vi "SaccadeAnalyser - Main.vi"(8 "error in (no error)":errorcluster, 11 "Data IN":T3={"Impulse Positions"=[{"Start"=5471, "End"=5813, "Impulse Plane"=enum."Yaw", "Impulse Direction +ve?"=FALSE, "Time offset"=0, "Amplitude offset"=0.0}, {"Start"=6974, "End"=7325, "Impulse Plane"=enum."Yaw", "Impulse Direction +ve?"=TRUE, "Time offset"=0, "Amplitude offset"=0.0}, {"Start"=7641, "End"=7980, "Impulse Plane"=enum."Yaw", "Impulse Direction +ve?"=FALSE, "Time offset"=0, "Amplitude offset"=0.0}, {"Start"=9060, "End"=9400, "Impulse Plane"=enum."Yaw", "Impulse Direction +ve?"=FALSE, "Time offset"=0, "Amplitude offset"=0.0}, {"Start"=9938, "End"=10282, "Impulse Plane"=enum."Yaw", "Impulse Direction +ve?"=FALSE, "Time offset"=0, "Amplitude offset"=0.0}, {"Start"=10800, "End"=11142, "Impulse Plane"=enum."Yaw", "Impulse Direction +ve?"=FALSE, "Time offset"=0, "Amplitude offset"=0.0}, {"Start"=11602, "End"=11942, "Impulse Plane"=enum."Yaw", "Impulse Direction +ve?"=TRUE, "Time offset"=0, "Amplitude offset"=0.0}, {"Start"=12449, "End"=12790, "Impulse Plane"=enum."Yaw", "Impulse Direction +ve?"=TRUE, "Time offset"=0, "Amplitude offset"=0.0}, {"Start"=13310, "End"=13653, "Impulse Plane"=enum."Yaw", "Impulse Direction +ve?"=TRUE, "Time offset"=0, "Amplitude offset"=0.0}, {"Start"=14191, "End"=14535, "Impulse Plane"=enum."Yaw", "Impulse Direction +ve?"=TRUE, "Time offset"=0, "Amplitude offset"=0.0}, {"Start"=15040, "End"=15380, "Impulse Plane"=enum."Yaw", "Impulse Direction +ve?"=FALSE, "Time offset"=0, "Amplitude offset"=0.0}, {"Start"=16780, "End"=17124, "Impulse Plane"=enum."Yaw", "Impulse Direction +ve?"=TRUE, "Time offset"=0, "Amplitude offset"=0.0}, {"Start"=17572, "End"=17913, "Impulse Plane"=enum."Yaw", "Impulse Direction +ve?"=FALSE, "Time offset"=0, "Amplitude offset"=0.0}, {"Start"=18369, "End"=18713, "Impulse Plane"=enum."Yaw", "Impulse Direction +ve?"=FALSE, "Time offset"=0, "Amplitude offset"=0.0}, {"Start"=19174, "End"=19519, "Impulse Plane"=enum."Yaw", "Impulse Direction +ve?"=FALSE, "Time offset"=0, "Amplitude offset"=0.0}, {"Start"=19928, "End"=20270, "Impulse Plane"=enum."Yaw", "Impulse Direction +ve?"=TRUE, "Time offset"=0, "Amplitude offset"=0.0}, {"Start"=20762, "End"=21121, "Impulse Plane"=enum."Yaw", "Impulse Direction +ve?"=FALSE, "Time offset"=0, "Amplitude offset"=0.0}, {"Start"=21554, "End"=21888, "Impulse Plane"=enum."Yaw", "Impulse Direction +ve?"=FALSE, "Time offset"=0, "Amplitude offset"=0.0}, {"Start"=22293, "End"=22639, "Impulse Plane"=enum."Yaw", "Impulse Direction +ve?"=TRUE, "Time offset"=0, "Amplitude offset"=0.0}, {"Start"=23109, "End"=23464, "Impulse Plane"=enum."Yaw", "Impulse Direction +ve?"=TRUE, "Time offset"=0, "Amplitude offset"=0.0}, {"Start"=23868, "End"=24215, "Impulse Plane"=enum."Yaw", "Impulse Direction +ve?"=TRUE, "Time offset"=0, "Amplitude offset"=0.0}, {"Start"=24643, "End"=24992, "Impulse Plane"=enum."Yaw", "Impulse Direction +ve?"=FALSE, "Time offset"=0, "Amplitude offset"=0.0}, {"Start"=25685, "End"=26023, "Impulse Plane"=enum."Yaw", "Impulse Direction +ve?"=FALSE, "Time offset"=0, "Amplitude offset"=0.0}, {"Start"=26431, "End"=26768, "Impulse Plane"=enum."Yaw", "Impulse Direction +ve?"=FALSE, "Time offset"=0, "Amplitude offset"=0.0}, {"Start"=27251, "End"=27595, "Impulse Plane"=enum."Yaw", "Impulse Direction +ve?"=FALSE, "Time offset"=0, "Amplitude offset"=0.0}, {"Start"=28832, "End"=29180, "Impulse Plane"=enum."Yaw", "Impulse Direction +ve?"=TRUE, "Time offset"=0, "Amplitude offset"=0.0}, {"Start"=31028, "End"=31383, "Impulse Plane"=enum."LARP", "Impulse Direction +ve?"=FALSE, "Time offset"=0, "Amplitude offset"=0.0}, {"Start"=32603, "End"=32936, "Impulse Plane"=enum."LARP", "Impulse Direction +ve?"=TRUE, "Time offset"=0, "Amplitude offset"=0.0}, {"Start"=33445, "End"=33779, "Impulse Plane"=enum."LARP", "Impulse Direction +ve?"=TRUE, "Time offset"=0, "Amplitude offset"=0.0}, {"Start"=34276, "End"=34629, "Impulse Plane"=enum."LARP", "Impulse Direction +ve?"=FALSE, "Time offset"=0, "Amplitude offset"=0.0}, {"Start"=35114, "End"=35460, "Impulse Plane"=enum."LARP", "Impulse Direction +ve?"=FALSE, "Time offset"=0, "Amplitude offset"=0.0}, {"Start"=35981, "End"=36324, "Impulse Plane"=enum."LARP", "Impulse Direction +ve?"=TRUE, "Time offset"=0, "Amplitude offset"=0.0}, {"Start"=36920, "End"=37249, "Impulse Plane"=enum."LARP", "Impulse Direction +ve?"=TRUE, "Time offset"=0, "Amplitude offset"=0.0}, {"Start"=37988, "End"=38322, "Impulse Plane"=enum."LARP", "Impulse Direction +ve?"=TRUE, "Time offset"=0, "Amplitude offset"=0.0}, {"Start"=38964, "End"=39324, "Impulse Plane"=enum."LARP", "Impulse Direction +ve?"=FALSE, "Time offset"=0, "Amplitude offset"=0.0}, {"Start"=39948, "End"=40284, "Impulse Plane"=enum."LARP", "Impulse Direction +ve?"=TRUE, "Time offset"=0, "Amplitude offset"=0.0}, {"Start"=40958, "End"=41293, "Impulse Plane"=enum."LARP", "Impulse Direction +ve?"=TRUE, "Time offset"=0, "Amplitude offset"=0.0}, {"Start"=41899, "End"=42229, "Impulse Plane"=enum."LARP", "Impulse Direction +ve?"=TRUE, "Time offset"=0, "Amplitude offset"=0.0}, {"Start"=42801, "End"=43154, "Impulse Plane"=enum."LARP", "Impulse Direction +ve?"=FALSE, "Time offset"=0, "Amplitude offset"=0.0}, {"Start"=43641, "End"=43980, "Impulse Plane"=enum."LARP", "Impulse Direction +ve?"=TRUE, "Time offset"=0, "Amplitude offset"=0.0}, {"Start"=44466, "End"=44821, "Impulse Plane"=enum."LARP", "Impulse Direction +ve?"=FALSE, "Time offset"=0, "Amplitude offset"=0.0}, {"Start"=45388, "End"=45722, "Impulse Plane"=enum."LARP", "Impulse Direction +ve?"=TRUE, "Time offset"=0, "Amplitude offset"=0.0}, {"Start"=46149, "End"=46510, "Impulse Plane"=enum."LARP", "Impulse Direction +ve?"=FALSE, "Time offset"=0, "Amplitude offset"=0.0}, {"Start"=47874, "End"=48206, "Impulse Plane"=enum."LARP", "Impulse Direction +ve?"=TRUE, "Time offset"=0, "Amplitude offset"=0.0}, {"Start"=50143, "End"=50479, "Impulse Plane"=enum."RALP", "Impulse Direction +ve?"=TRUE, "Time offset"=0, "Amplitude offset"=0.0}, {"Start"=50976, "End"=51310, "Impulse Plane"=enum."RALP", "Impulse Direction +ve?"=FALSE, "Time offset"=0, "Amplitude offset"=0.0}, {"Start"=51892, "End"=52226, "Impulse Plane"=enum."RALP", "Impulse Direction +ve?"=FALSE, "Time offset"=0, "Amplitude offset"=0.0}, {"Start"=52839, "End"=53171, "Impulse Plane"=enum."RALP", "Impulse Direction +ve?"=FALSE, "Time offset"=0, "Amplitude offset"=0.0}, {"Start"=53676, "End"=54012, "Impulse Plane"=enum."RALP", "Impulse Direction +ve?"=TRUE, "Time offset"=0, "Amplitude offset"=0.0}, {"Start"=54530, "End"=54877, "Impulse Plane"=enum."RALP", "Impulse Direction +ve?"=FALSE, "Time offset"=0, "Amplitude offset"=0.0}, {"Start"=55371, "End"=55711, "Impulse Plane"=enum."RALP", "Impulse Direction +ve?"=TRUE, "Time offset"=0, "Amplitude offset"=0.0}, {"Start"=56153, "End"=56482, "Impulse Plane"=enum."RALP", "Impulse Direction +ve?"=FALSE, "Time offset"=0, "Amplitude offset"=0.0}, {"Start"=57053, "End"=57390, "Impulse Plane"=enum."RALP", "Impulse Direction +ve?"=FALSE, "Time offset"=0, "Amplitude offset"=0.0}, {"Start"=57954, "End"=58292, "Impulse Plane"=enum."RALP", "Impulse Direction +ve?"=FALSE, "Time offset"=0, "Amplitude offset"=0.0}, {"Start"=58794, "End"=59130, "Impulse Plane"=enum."RALP", "Impulse Direction +ve?"=TRUE, "Time offset"=0, "Amplitude offset"=0.0}, {"Start"=59587, "End"=59931, "Impulse Plane"=enum."RALP", "Impulse Direction +ve?"=TRUE, "Time offset"=0, "Amplitude offset"=0.0}, {"Start"=60399, "End"=60744, "Impulse Plane"=enum."RALP", "Impulse Direction +ve?"=FALSE, "Time offset"=0, "Amplitude offset"=0.0}, {"Start"=61218, "End"=61559, "Impulse Plane"=enum."RALP", "Impulse Direction +ve?"=FALSE, "Time offset"=0, "Amplitude offset"=0.0}, {"Start"=62100, "End"=62442, "Impulse Plane"=enum."RALP", "Impulse Direction +ve?"=FALSE, "Time offset"=0, "Amplitude offset"=0.0}, {"Start"=62989, "End"=63322, "Impulse Plane"=enum."RALP", "Impulse Direction +ve?"=FALSE, "Time offset"=0, "Amplitude offset"=0.0}, {"Start"=63787, "End"=64136, "Impulse Plane"=enum."RALP", "Impulse Direction +ve?"=TRUE, "Time offset"=0, "Amplitude offset"=0.0}, {"Start"=64603, "End"=64953, "Impulse Plane"=enum."RALP", "Impulse Direction +ve?"=FALSE, "Time offset"=0, "Amplitude offset"=0.0}, {"Start"=65462, "End"=65795, "Impulse Plane"=enum."RALP", "Impulse Direction +ve?"=FALSE, "Time offset"=0, "Amplitude offset"=0.0}, {"Start"=66308, "End"=66645, "Impulse Plane"=enum."RALP", "Impulse Direction +ve?"=FALSE, "Time offset"=0, "Amplitude offset"=0.0}, {"Start"=67052, "End"=67402, "Impulse Plane"=enum."RALP", "Impulse Direction +ve?"=TRUE, "Time offset"=0, "Amplitude offset"=0.0}], "No. Imp"=15, "Parameter Time Series"=[{"time offset"=0.0, "Offset"=0.0, "Gain"=1.0, "inverse"=FALSE, "filter data"=FALSE, "dots"=FALSE, "interpolate"=FALSE, "List 1"=5, "Color Box"=6618880, "Boolean"=TRUE}, {"time offset"=0.0, "Offset"=0.0, "Gain"=1.0, "inverse"=FALSE, "filter data"=FALSE, "dots"=FALSE, "interpolate"=FALSE, "List 1"=6, "Color Box"=6618880, "Boolean"=FALSE}, {"time offset"=0.0, "Offset"=0.0, "Gain"=1.0, "inverse"=FALSE, "filter data"=FALSE, "dots"=FALSE, "interpolate"=FALSE, "List 1"=7, "Color Box"=6618880, "Boolean"=FALSE}, {"time offset"=0.0, "Offset"=0.0, "Gain"=1.0, "inverse"=FALSE, "filter data"=FALSE, "dots"=FALSE, "interpolate"=FALSE, "List 1"=13, "Color Box"=16777224, "Boolean"=TRUE}, {"time offset"=0.0, "Offset"=0.0, "Gain"=1.0, "inverse"=FALSE, "filter data"=FALSE, "dots"=FALSE, "interpolate"=FALSE, "List 1"=14, "Color Box"=16777224, "Boolean"=FALSE}, {"time offset"=0.0, "Offset"=0.0, "Gain"=1.0, "inverse"=FALSE, "filter data"=FALSE, "dots"=FALSE, "interpolate"=FALSE, "List 1"=15, "Color Box"=16777224, "Boolean"=FALSE}], "Parameter Impuls Series"=[{"Color"=6618880, "Visible"=TRUE, "Channel"=1, "Invert"=FALSE, "Desaccade"=FALSE, "Offset"=0.0, "Gain"=1.0}, {"Color"=6618880, "Visible"=FALSE, "Channel"=6, "Invert"=FALSE, "Desaccade"=FALSE, "Offset"=0.0, "Gain"=1.0}, {"Color"=6618880, "Visible"=FALSE, "Channel"=7, "Invert"=FALSE, "Desaccade"=FALSE, "Offset"=0.0, "Gain"=1.0}, {"Color"=16777224, "Visible"=TRUE, "Channel"=13, "Invert"=FALSE, "Desaccade"=FALSE, "Offset"=0.0, "Gain"=1.0}, {"Color"=16777224, "Visible"=FALSE, "Channel"=14, "Invert"=FALSE, "Desaccade"=FALSE, "Offset"=0.0, "Gain"=1.0}, {"Color"=16777224, "Visible"=FALSE, "Channel"=15, "Invert"=FALSE, "Desaccade"=FALSE, "Offset"=0.0, "Gain"=1.0}], "Experiment Parameters"={"Freq"=0.0, "Vel"=0, "Acc"=0, "Stimulus"="Head Impulse"}, "Autosort File"=refnum, "Data File"={"Data Channels"=array34x71049[2415666 elements], "Sample Rate"=500, "Channel List"=["Hz Position-in-Head", "Hz Velocity-in-Head", "Hy Position-in-Head", "Hy Velocity-in-Head", "Hx Position-in-Head", "Hx Velocity-in-Head", "Hl Velocity-in-Head", "Hr Velocity-in-Head", "Lx Position-in-Head", "Ly Position-in-Head", "Lz Position-in-Head", "Lx Velocity-in-Head", "Ly Velocity-in-Head", "Lz Velocity-in-Head", "Ll Velocity-in-Head", "Lr Velocity-in-Head", "Rx Position-in-Head", "Ry Position-in-Head", "Rz Position-in-Head", "Rx Velocity-in-Head", "Ry Velocity-in-Head", "Rz Velocity-in-Head", "Rl Velocity-in-Head", "Rr Velocity-in-Head", "Target on/off", "aux input 1", "aux input 2", " ", "", "", "", "Target Hor", "Target Ver", ""]}, "Experiment data path"=path "C:/Users/w.figtree/Desktop/Coils Data/3", "Image data path"=path "/Macintosh HD/Users/patrick/Studium/Diploma Thesis/Data Analysis", "LVS data path"=path "/Macintosh HD/Users/patrick/Studium/Diploma Thesis/Data Analysis", "Raw copy path"=path "/Macintosh HD/Users/patrick/Studium/Diploma Thesis/Data Analysis", "filename"="passive_lvs.lvs", "desaccading parameters"={"Tolerance"=3, "Acc Range"=7000.0, "Sample Rate"=500, "Impulse Plane 2"=enum."Yaw", "Impulse dir"=FALSE}, "Experiment Parameters 2"={"Subject"="SE Trial Short Term", "Strain"="", "Rotation plane"="", "Experimenter"=" ", "Trial"=0.0, "Time"=0.0}, "Excel"={"Excel._Application"=refnum, "Use Excel"=TRUE, "Worksheet SINE"=refnum, "Row SINE"=0, "Worksheet TRANS"=refnum, "Row TRANS"=0}, "Session Config File"=refnum, "Autosort Parameter Set"=4, "EMA Version"="EMA 2016a", "desacc "={"Threshold 1 [Acc]"=7000.0, "Threshold 2 [% of TH1]"=60, "tolerance"=3, "Search WD "=0.1, " always use TH2"=FALSE, "Range"=3.0, "Max time"=120.0, "Min time"=20.0, "Velocity Threshold"=150}, "Cycle Nr for Saccades"={"POS"=0, "NEG"=0}, "calibration name"="u_calibration_1_p00001s001_calib.mat", "Excel"=refnum} {"Parameter Time Series"."time offset" format="%.3f"; "Parameter Time Series"."Gain" format="%.1f"; "Parameter Time Series"."Offset" format="%.1f"; "Parameter Time Series"."List 1" items=["Motor-Pos", "Motor-Vel", "Lx Position-in-Head", "Ly Position-in-Head", "Lz Position-in-Head", "Lx Velocity-in-Head", "Ly Velocity-in-Head", "Lz Velocity-in-Head", "Ll Velocity-in-Head", "Lr Velocity-in-Head", "Lx Accel-in-Head", "Ly Accel-in-Head", "Lz Accel-in-Head", "Rx Position-in-Head", "Ry Position-in-Head", "Rz Position-in-Head", "Rx Velocity-in-Head", "Ry Velocity-in-Head", "Rz Velocity-in-Head", "Rl Velocity-in-Head", "Rr Velocity-in-Head", "Rx Accel-in-Head", "Ry Accel-in-Head", "Rz Accel-in-Head", "Global Trigger", "", "", ""]; "Parameter Impuls Series"."Gain" format="%.1f"; "Parameter Impuls Series"."Offset" format="%.1f"}) -> (0 "error out":errorcluster, 3 "Data OUT":T3={"Impulse Positions"=[{"Start"=5471, "End"=5813, "Impulse Plane"=enum."Yaw", "Impulse Direction +ve?"=FALSE, "Time offset"=0, "Amplitude offset"=0.0}, {"Start"=6974, "End"=7325, "Impulse Plane"=enum."Yaw", "Impulse Direction +ve?"=TRUE, "Time offset"=0, "Amplitude offset"=0.0}, {"Start"=7641, "End"=7980, "Impulse Plane"=enum."Yaw", "Impulse Direction +ve?"=FALSE, "Time offset"=0, "Amplitude offset"=0.0}, {"Start"=9060, "End"=9400, "Impulse Plane"=enum."Yaw", "Impulse Direction +ve?"=FALSE, "Time offset"=0, "Amplitude offset"=0.0}, {"Start"=9938, "End"=10282, "Impulse Plane"=enum."Yaw", "Impulse Direction +ve?"=FALSE, "Time offset"=0, "Amplitude offset"=0.0}, {"Start"=10800, "End"=11142, "Impulse Plane"=enum."Yaw", "Impulse Direction +ve?"=FALSE, "Time offset"=0, "Amplitude offset"=0.0}, {"Start"=11602, "End"=11942, "Impulse Plane"=enum."Yaw", "Impulse Direction +ve?"=TRUE, "Time offset"=0, "Amplitude offset"=0.0}, {"Start"=12449, "End"=12790, "Impulse Plane"=enum."Yaw", "Impulse Direction +ve?"=TRUE, "Time offset"=0, "Amplitude offset"=0.0}, {"Start"=13310, "End"=13653, "Impulse Plane"=enum."Yaw", "Impulse Direction +ve?"=TRUE, "Time offset"=0, "Amplitude offset"=0.0}, {"Start"=14191, "End"=14535, "Impulse Plane"=enum."Yaw", "Impulse Direction +ve?"=TRUE, "Time offset"=0, "Amplitude offset"=0.0}, {"Start"=15040, "End"=15380, "Impulse Plane"=enum."Yaw", "Impulse Direction +ve?"=FALSE, "Time offset"=0, "Amplitude offset"=0.0}, {"Start"=16780, "End"=17124, "Impulse Plane"=enum."Yaw", "Impulse Direction +ve?"=TRUE, "Time offset"=0, "Amplitude offset"=0.0}, {"Start"=17572, "End"=17913, "Impulse Plane"=enum."Yaw", "Impulse Direction +ve?"=FALSE, "Time offset"=0, "Amplitude offset"=0.0}, {"Start"=18369, "End"=18713, "Impulse Plane"=enum."Yaw", "Impulse Direction +ve?"=FALSE, "Time offset"=0, "Amplitude offset"=0.0}, {"Start"=19174, "End"=19519, "Impulse Plane"=enum."Yaw", "Impulse Direction +ve?"=FALSE, "Time offset"=0, "Amplitude offset"=0.0}, {"Start"=19928, "End"=20270, "Impulse Plane"=enum."Yaw", "Impulse Direction +ve?"=TRUE, "Time offset"=0, "Amplitude offset"=0.0}, {"Start"=20762, "End"=21121, "Impulse Plane"=enum."Yaw", "Impulse Direction +ve?"=FALSE, "Time offset"=0, "Amplitude offset"=0.0}, {"Start"=21554, "End"=21888, "Impulse Plane"=enum."Yaw", "Impulse Direction +ve?"=FALSE, "Time offset"=0, "Amplitude offset"=0.0}, {"Start"=22293, "End"=22639, "Impulse Plane"=enum."Yaw", "Impulse Direction +ve?"=TRUE, "Time offset"=0, "Amplitude offset"=0.0}, {"Start"=23109, "End"=23464, "Impulse Plane"=enum."Yaw", "Impulse Direction +ve?"=TRUE, "Time offset"=0, "Amplitude offset"=0.0}, {"Start"=23868, "End"=24215, "Impulse Plane"=enum."Yaw", "Impulse Direction +ve?"=TRUE, "Time offset"=0, "Amplitude offset"=0.0}, {"Start"=24643, "End"=24992, "Impulse Plane"=enum."Yaw", "Impulse Direction +ve?"=FALSE, "Time offset"=0, "Amplitude offset"=0.0}, {"Start"=25685, "End"=26023, "Impulse Plane"=enum."Yaw", "Impulse Direction +ve?"=FALSE, "Time offset"=0, "Amplitude offset"=0.0}, {"Start"=26431, "End"=26768, "Impulse Plane"=enum."Yaw", "Impulse Direction +ve?"=FALSE, "Time offset"=0, "Amplitude offset"=0.0}, {"Start"=27251, "End"=27595, "Impulse Plane"=enum."Yaw", "Impulse Direction +ve?"=FALSE, "Time offset"=0, "Amplitude offset"=0.0}, {"Start"=28832, "End"=29180, "Impulse Plane"=enum."Yaw", "Impulse Direction +ve?"=TRUE, "Time offset"=0, "Amplitude offset"=0.0}, {"Start"=31028, "End"=31383, "Impulse Plane"=enum."LARP", "Impulse Direction +ve?"=FALSE, "Time offset"=0, "Amplitude offset"=0.0}, {"Start"=32603, "End"=32936, "Impulse Plane"=enum."LARP", "Impulse Direction +ve?"=TRUE, "Time offset"=0, "Amplitude offset"=0.0}, {"Start"=33445, "End"=33779, "Impulse Plane"=enum."LARP", "Impulse Direction +ve?"=TRUE, "Time offset"=0, "Amplitude offset"=0.0}, {"Start"=34276, "End"=34629, "Impulse Plane"=enum."LARP", "Impulse Direction +ve?"=FALSE, "Time offset"=0, "Amplitude offset"=0.0}, {"Start"=35114, "End"=35460, "Impulse Plane"=enum."LARP", "Impulse Direction +ve?"=FALSE, "Time offset"=0, "Amplitude offset"=0.0}, {"Start"=35981, "End"=36324, "Impulse Plane"=enum."LARP", "Impulse Direction +ve?"=TRUE, "Time offset"=0, "Amplitude offset"=0.0}, {"Start"=36920, "End"=37249, "Impulse Plane"=enum."LARP", "Impulse Direction +ve?"=TRUE, "Time offset"=0, "Amplitude offset"=0.0}, {"Start"=37988, "End"=38322, "Impulse Plane"=enum."LARP", "Impulse Direction +ve?"=TRUE, "Time offset"=0, "Amplitude offset"=0.0}, {"Start"=38964, "End"=39324, "Impulse Plane"=enum."LARP", "Impulse Direction +ve?"=FALSE, "Time offset"=0, "Amplitude offset"=0.0}, {"Start"=39948, "End"=40284, "Impulse Plane"=enum."LARP", "Impulse Direction +ve?"=TRUE, "Time offset"=0, "Amplitude offset"=0.0}, {"Start"=40958, "End"=41293, "Impulse Plane"=enum."LARP", "Impulse Direction +ve?"=TRUE, "Time offset"=0, "Amplitude offset"=0.0}, {"Start"=41899, "End"=42229, "Impulse Plane"=enum."LARP", "Impulse Direction +ve?"=TRUE, "Time offset"=0, "Amplitude offset"=0.0}, {"Start"=42801, "End"=43154, "Impulse Plane"=enum."LARP", "Impulse Direction +ve?"=FALSE, "Time offset"=0, "Amplitude offset"=0.0}, {"Start"=43641, "End"=43980, "Impulse Plane"=enum."LARP", "Impulse Direction +ve?"=TRUE, "Time offset"=0, "Amplitude offset"=0.0}, {"Start"=44466, "End"=44821, "Impulse Plane"=enum."LARP", "Impulse Direction +ve?"=FALSE, "Time offset"=0, "Amplitude offset"=0.0}, {"Start"=45388, "End"=45722, "Impulse Plane"=enum."LARP", "Impulse Direction +ve?"=TRUE, "Time offset"=0, "Amplitude offset"=0.0}, {"Start"=46149, "End"=46510, "Impulse Plane"=enum."LARP", "Impulse Direction +ve?"=FALSE, "Time offset"=0, "Amplitude offset"=0.0}, {"Start"=47874, "End"=48206, "Impulse Plane"=enum."LARP", "Impulse Direction +ve?"=TRUE, "Time offset"=0, "Amplitude offset"=0.0}, {"Start"=50143, "End"=50479, "Impulse Plane"=enum."RALP", "Impulse Direction +ve?"=TRUE, "Time offset"=0, "Amplitude offset"=0.0}, {"Start"=50976, "End"=51310, "Impulse Plane"=enum."RALP", "Impulse Direction +ve?"=FALSE, "Time offset"=0, "Amplitude offset"=0.0}, {"Start"=51892, "End"=52226, "Impulse Plane"=enum."RALP", "Impulse Direction +ve?"=FALSE, "Time offset"=0, "Amplitude offset"=0.0}, {"Start"=52839, "End"=53171, "Impulse Plane"=enum."RALP", "Impulse Direction +ve?"=FALSE, "Time offset"=0, "Amplitude offset"=0.0}, {"Start"=53676, "End"=54012, "Impulse Plane"=enum."RALP", "Impulse Direction +ve?"=TRUE, "Time offset"=0, "Amplitude offset"=0.0}, {"Start"=54530, "End"=54877, "Impulse Plane"=enum."RALP", "Impulse Direction +ve?"=FALSE, "Time offset"=0, "Amplitude offset"=0.0}, {"Start"=55371, "End"=55711, "Impulse Plane"=enum."RALP", "Impulse Direction +ve?"=TRUE, "Time offset"=0, "Amplitude offset"=0.0}, {"Start" (continued)
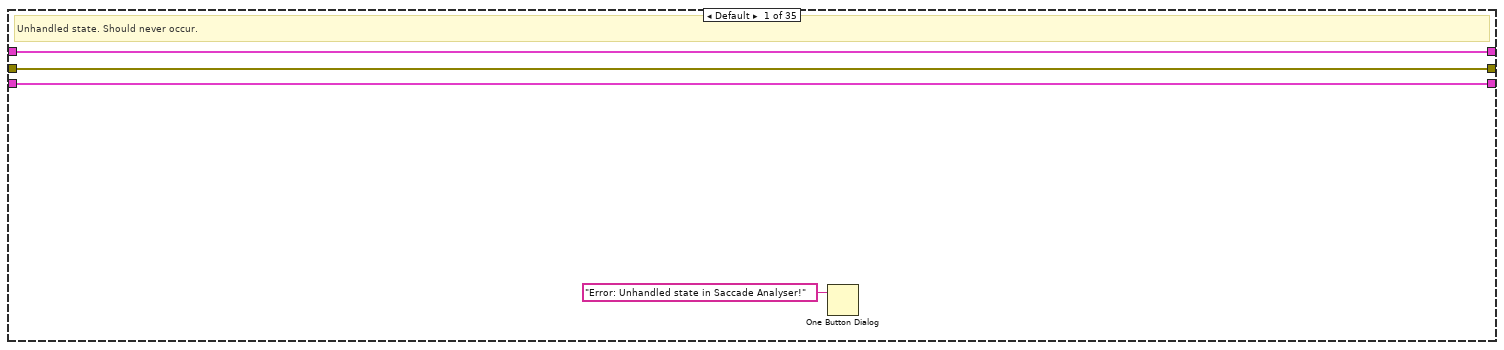
[diagram p2: hidden frame]
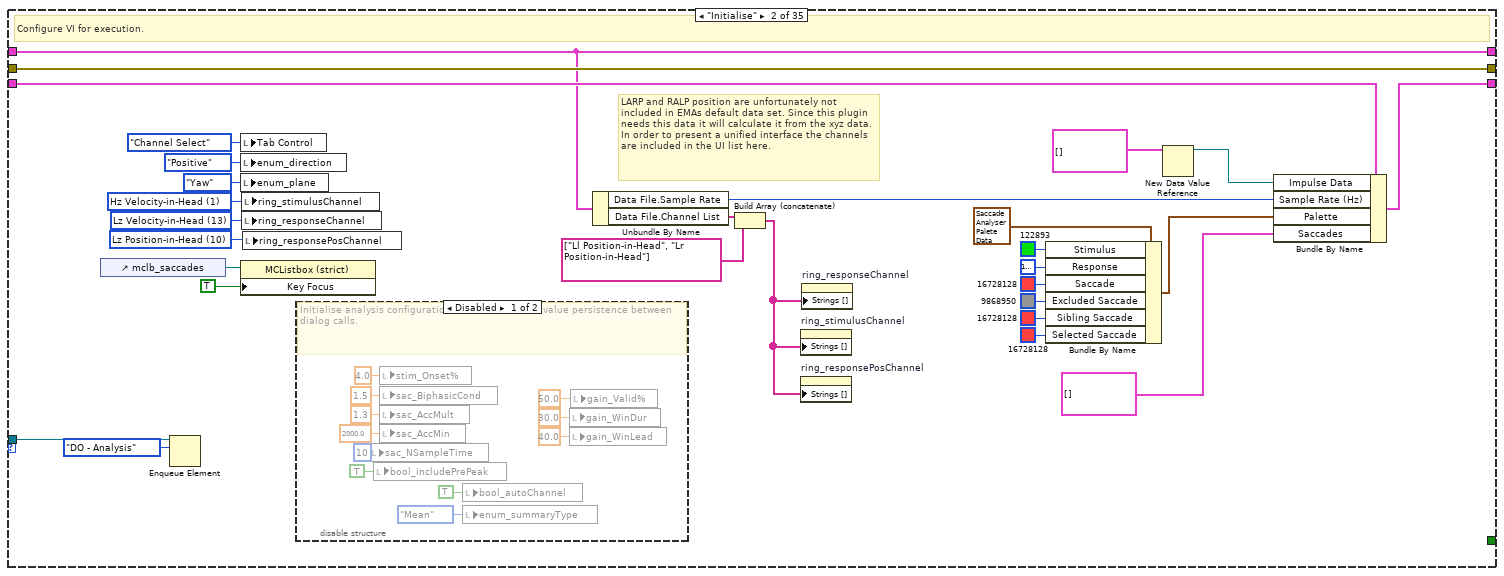
[diagram p3: hidden frame]
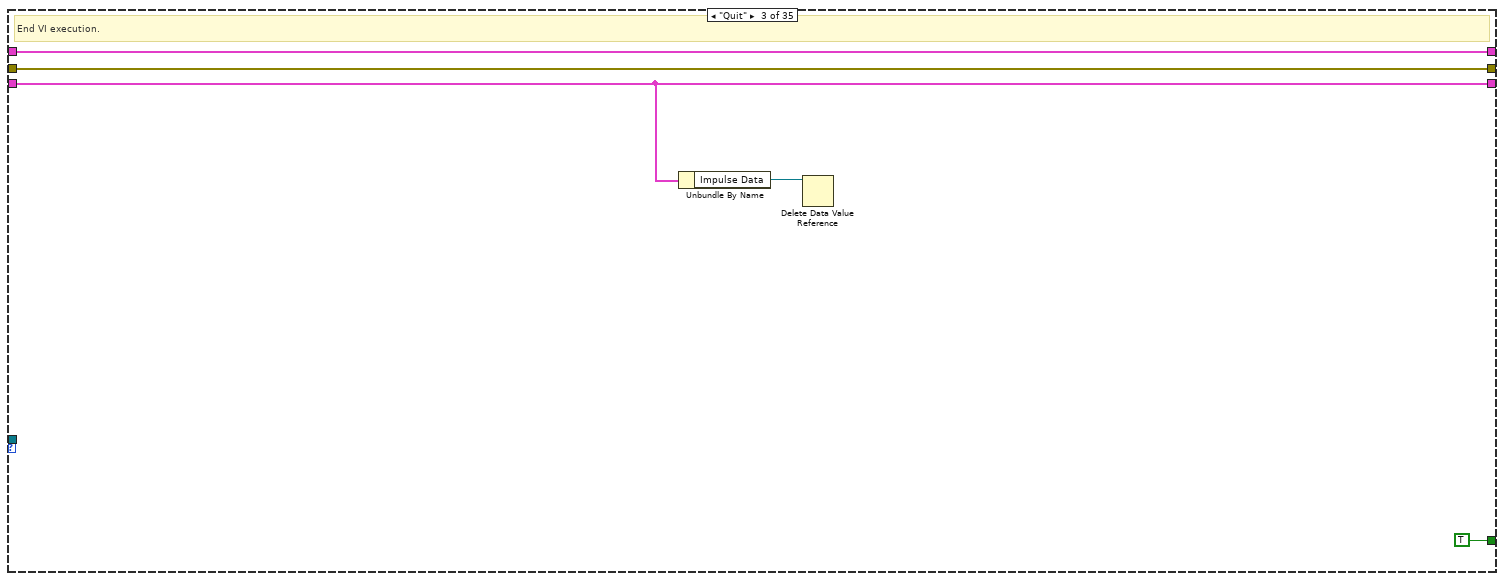
[diagram p5: hidden frame]
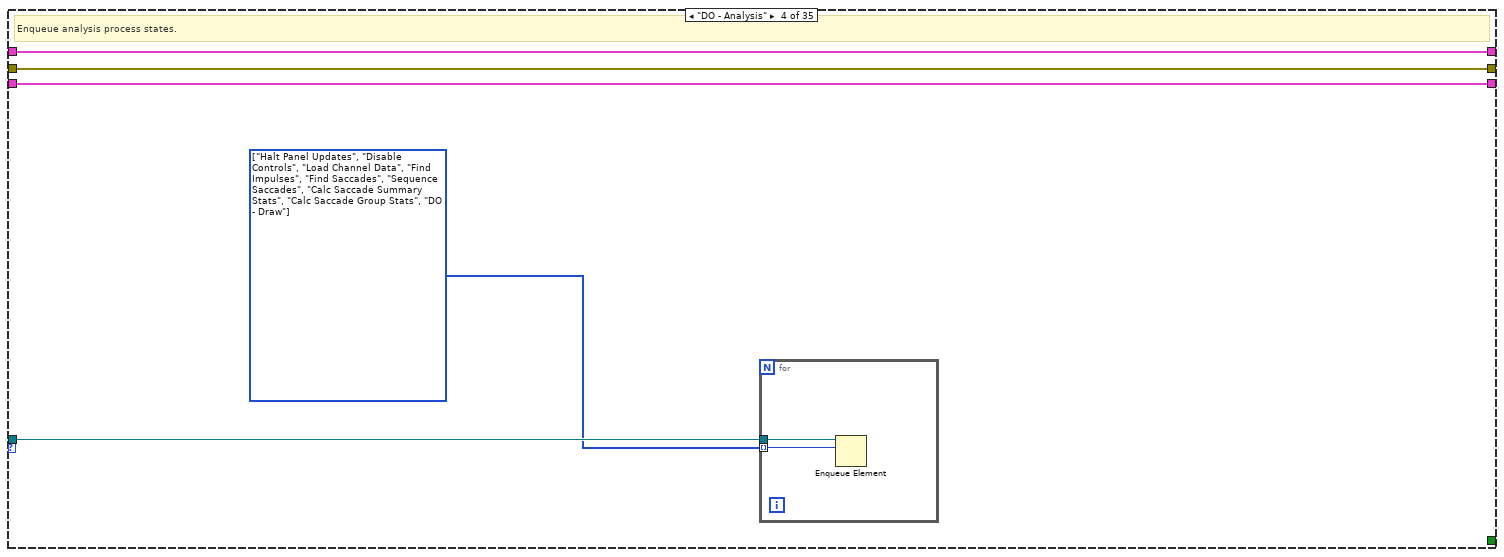
[diagram p6: hidden frame]
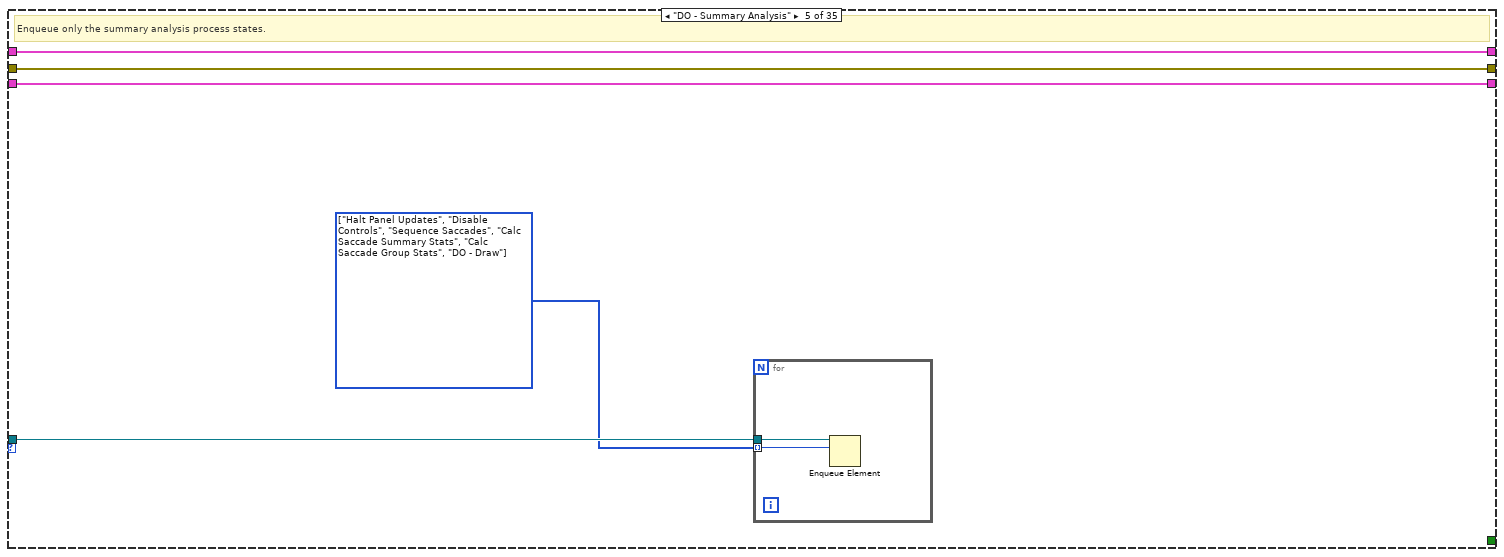
[diagram p7: hidden frame]
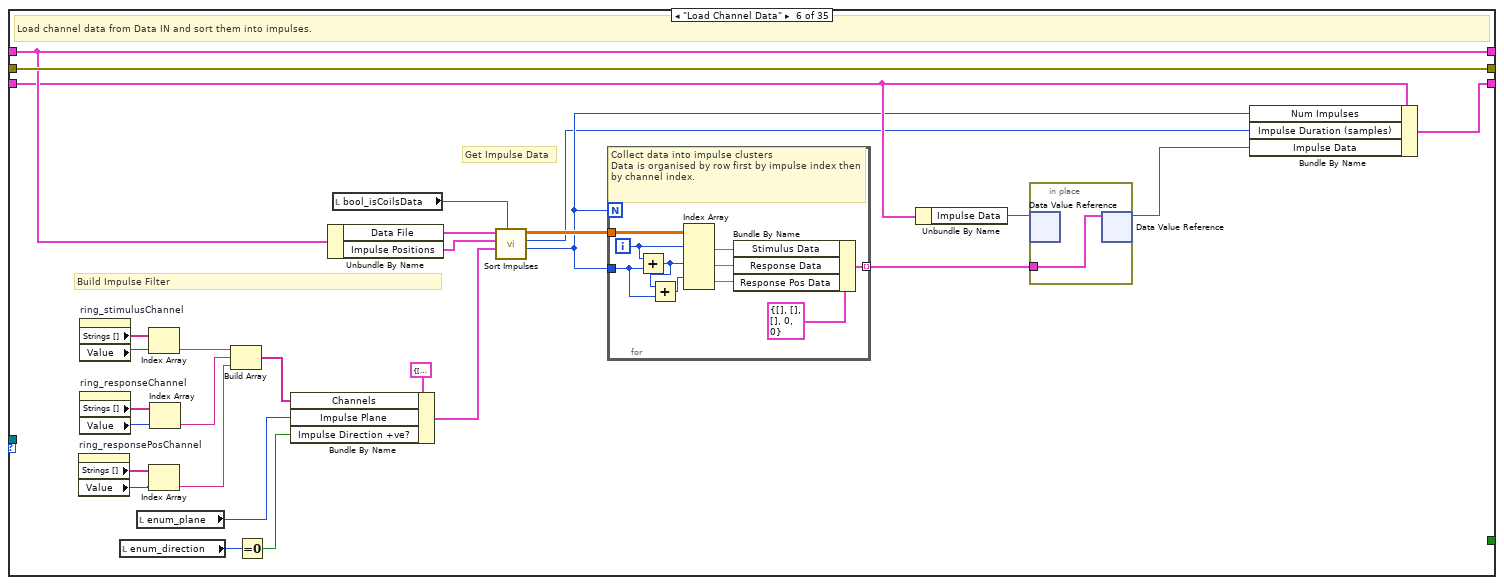
[diagram p8: hidden frame]
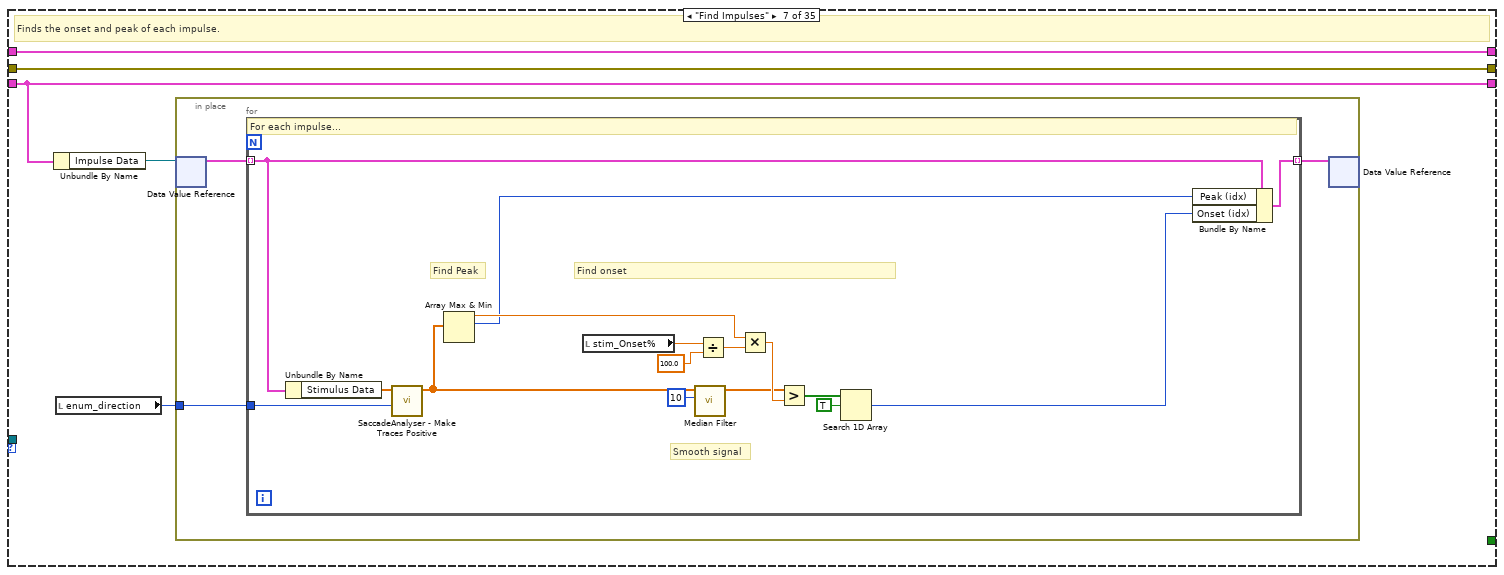
[diagram p9: hidden frame]
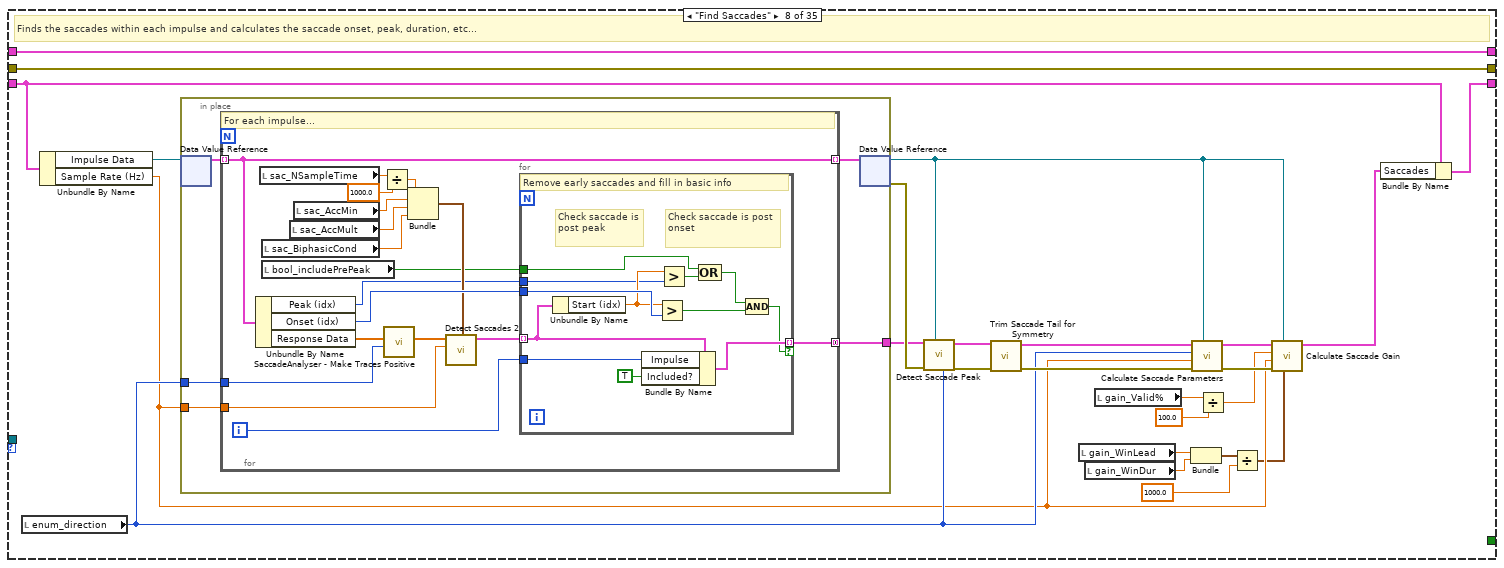
[diagram p10: hidden frame]
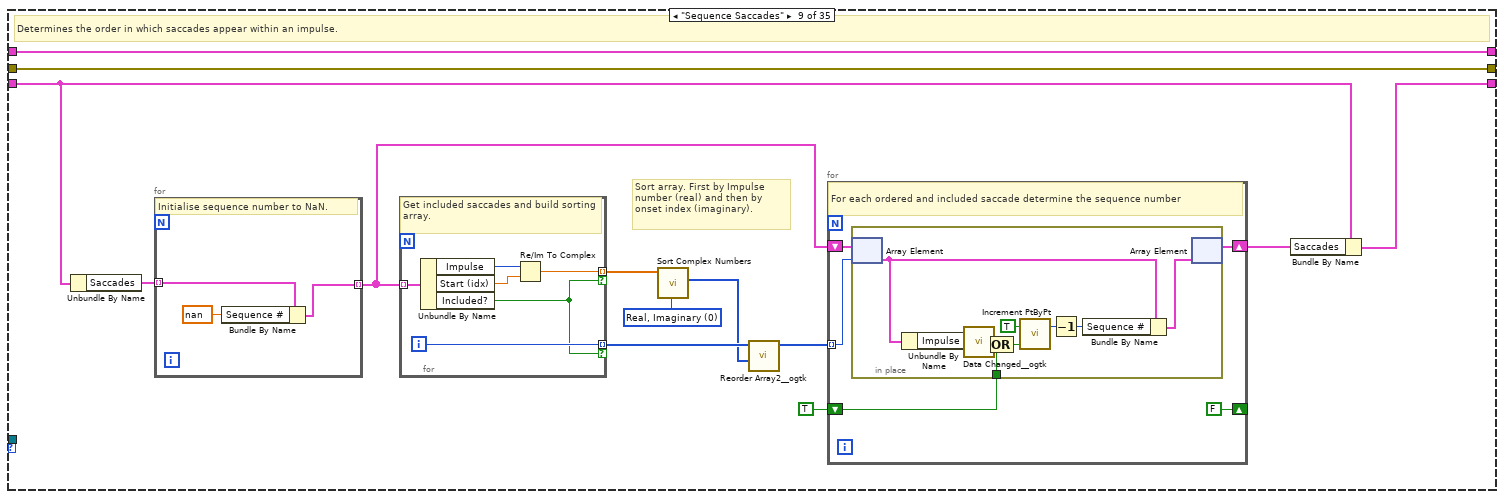
[diagram p11: hidden frame]
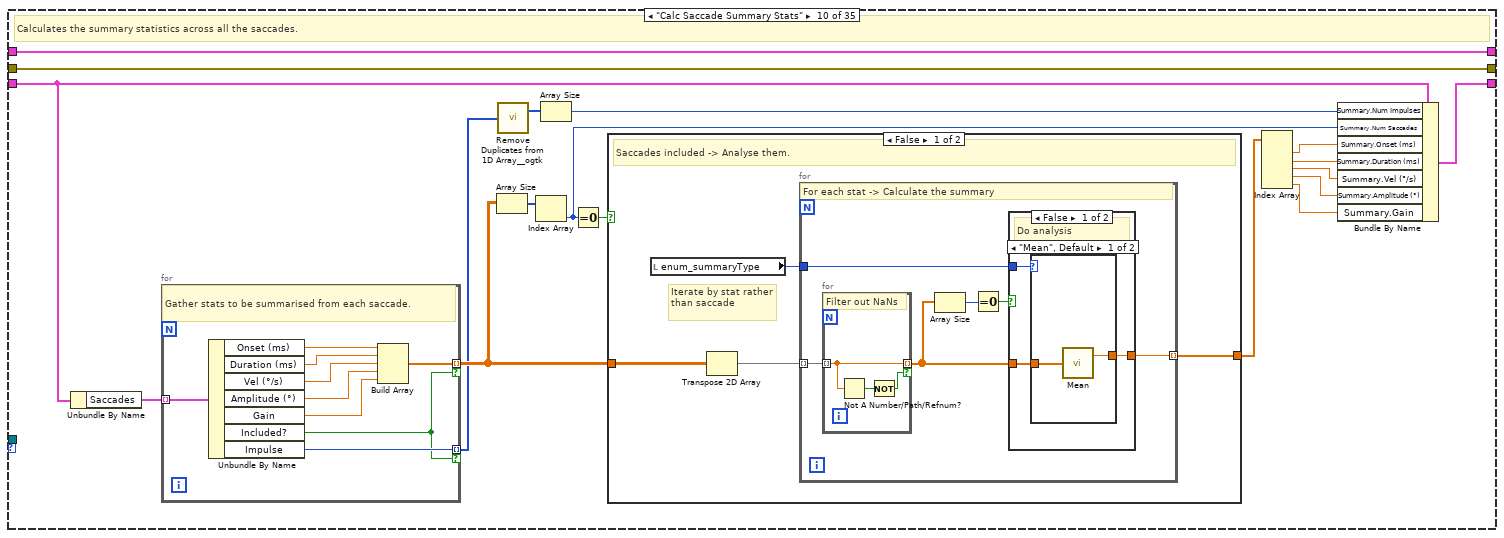
[diagram p12: hidden frame]
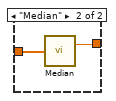
[diagram p13: hidden frame]
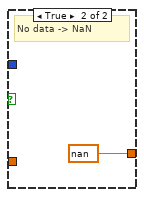
[diagram p14: hidden frame]
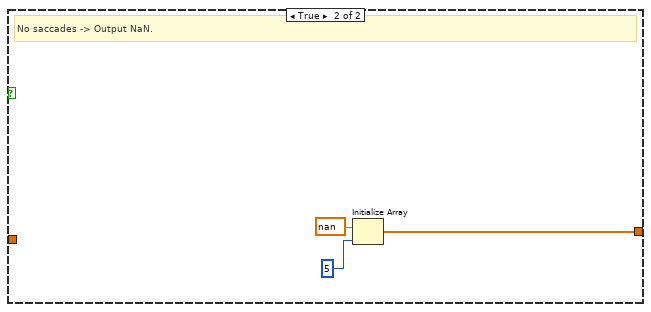
[diagram p15: hidden frame]
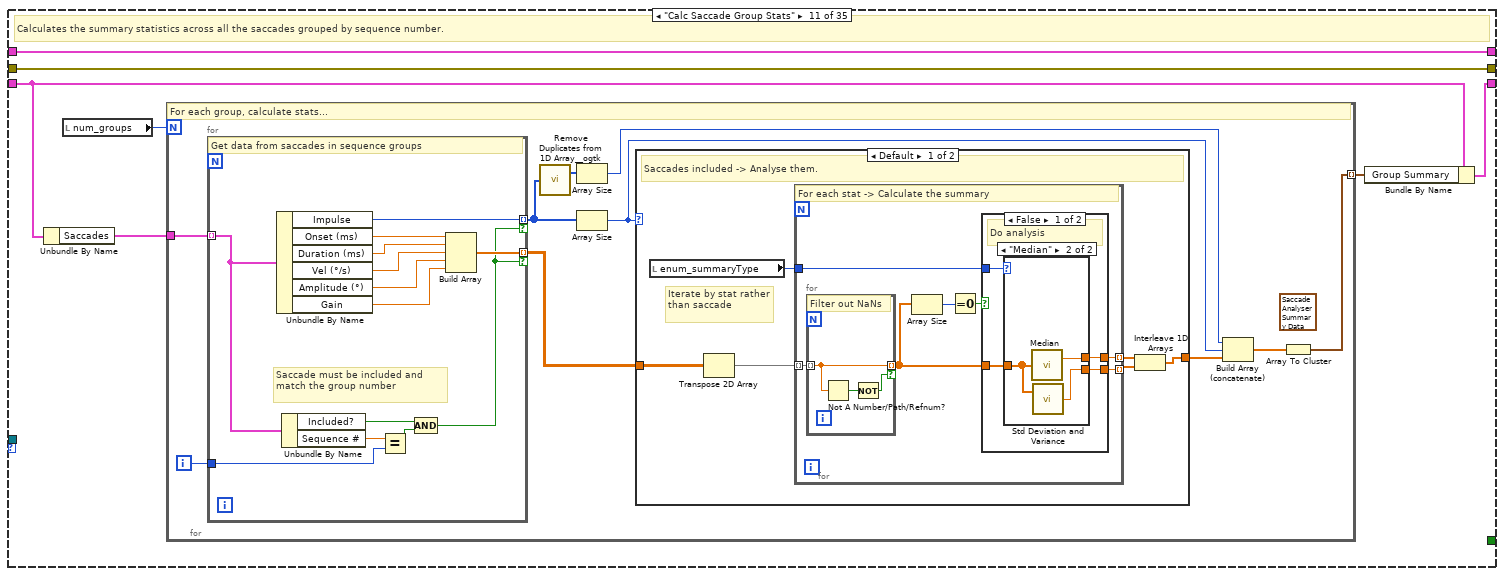
[diagram p16: hidden frame]
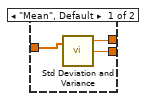
[diagram p17: hidden frame]
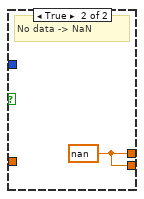
[diagram p18: hidden frame]
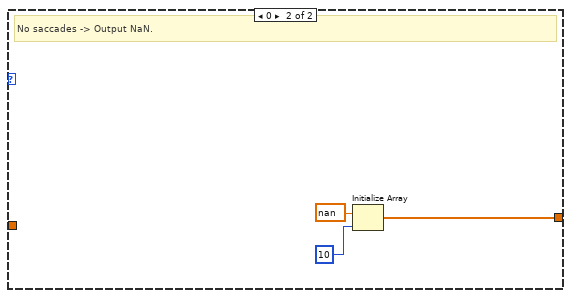
[diagram p19: hidden frame]
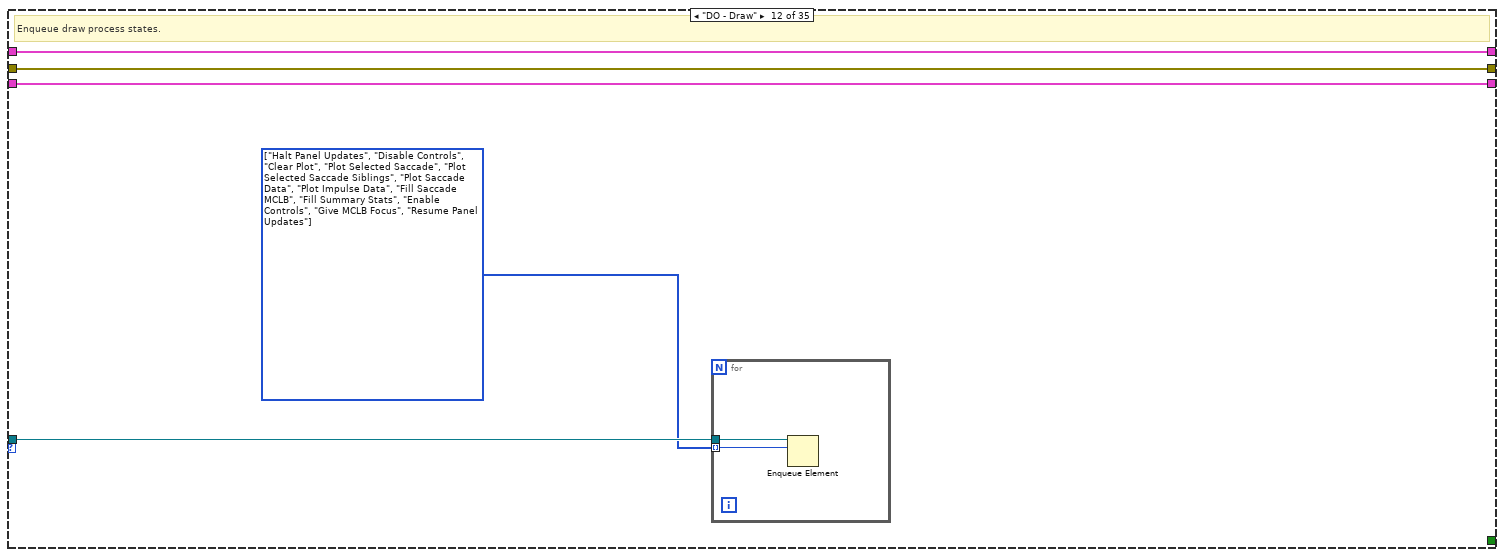
[diagram p20: hidden frame]
        n443 = Index Array(array=w802, index=w803) -> (element=w797:string)
        n444 = Index Array(array=w801, index=w800) -> (element=w796:string)
        n445 = call <userlib>:"Write.vi"("Cell (Append to next row)"=cluster{"Row":i32, "Col":i32} {"Row"=0, "Col"=0}, "Data"=w793, "Excel in"=w788) -> ("error out"=w807:errorcluster, "Excel out"=w808:refnum<class "Excel.lvclass">)  [unwired: 6 in, 1 out]
        n446 = Build Array(w799, w798, w797, w796) -> (w784:string[])
        n447 = Build Array (concatenate)(w784, w785) -> (w783:string[])
        n448 = call <userlib>:"Write.vi"("error in (no error)"=w807, "Data"=w783, "Excel in"=w808) -> ("error out"=w786:errorcluster, "Excel out"=w787:refnum<class "Excel.lvclass">)  [unwired: 6 in, 1 out]
        n449 = call <userlib>:"Save.vi"("error in (no error)"=w786, "Excel in"=w787) -> ("Excel out"=w806:refnum<class "Excel.lvclass">)  [unwired: 7 in, 2 out]
        n450 = Bundle By Name(cluster=w789, "Excel"=w806) -> (w790:T3)
      }
      frame "Export - Open Saccades" {
        # "Use provided sheet name or fall back to a default"
        # "Opens an Excel instance, workbook, and saccades worksheet."
        n451 = local read "export_SaccadesSheet"() -> (w835:string)
        n452 = Unbundle By Name(w829) -> ("Excel"=w832:refnum<class "Excel.lvclass">)
        n453 = Empty String/Path?(string/path=w835) -> (empty?=w836:bool)
        n454 = Select(t="Saccades", s=w836, f=w835) -> (s? t:f=w833:string)
        n455 = call <userlib>:"Open.vi"("Worksheet Name (Sheet1)"=w833, "Excel in"=w832) -> ("Excel out"=w831:refnum<class "Excel.lvclass">)  [unwired: 8 in, 1 out]
        n456 = Bundle By Name(cluster=w829, "Excel"=w831) -> (w830:T3)
      }
      frame "Export - Saccades" {
        # "Get common data"
        # "Save the workbook."
        # "Write header"
        # "Exports all saccade data to an open Excel sheet."
        n457 = Unbundle By Name(w840) -> ("Saccades"=w848:T8[], "Summary"=w847:T9, "Num Impulses"=w838:i32)
        n458 = Unbundle By Name(w839) -> ("Excel"=w842:refnum<class "Excel.lvclass">)
        n459 = Unbundle By Name(w847) -> ("Num Impulses"=w846:dbl, "Num Saccades"=w845:dbl)
        n460 = Unbundle By Name(w839) -> ("Experiment Parameters 2.Subject"=w857:string)
        n461 = property on="enum_plane" class="Enum (strict)"() -> ("Strings []"=w856:string[], "Value"=w855:T14)  [unwired: 2 in, 2 out]
        n462 = property on="enum_direction" class="Enum (strict)"() -> ("Strings []"=w853:string[], "Value"=w854:enum16{"Positive", "Negative"})  [unwired: 2 in, 2 out]
        n463 = Build Array(w838, w846, w845) -> (w844:dbl[])
        n464 = Index Array(array=w856, index=w855) -> (element=w852:string)
        n465 = Index Array(array=w853, index=w854) -> (element=w851:string)
        n466 = To Double Precision Float(number=w844) -> (double precision float=w843:dbl[])
        n467 = call <userlib>:"Write.vi"("Cell (Append to next row)"=cluster{"Row":i32, "Col":i32} {"Row"=0, "Col"=0}, "Data"=string[] ["Subject", "Plane", "Direction", "Total Impulses", "Num Impulses", "Num Saccades", "Impulse ID", "Sequence #", "Onset (ms)", "Duration (ms)", "Velocity (°/s)", "Amplitude (°)", "Gain"], "Excel in"=w842) -> ("error out"=w861:errorcluster, "Excel out"=w862:refnum<class "Excel.lvclass">)  [unwired: 6 in, 1 out]
        n468 = Build Array(w857, w852, w851) -> (w849:string[])
        n469 = for {
          shift-right: [w870] -> w860
          shift-left: w862 -> [w872]
          shift-right: [w869] -> w859
          shift-left: w861 -> [w871]
          tunnel: w849 -> [w867]
          tunnel: w848 -> [w866] mode=indexing
          tunnel: w843 -> [w865]
          # "Append data row for each saccade"
          n470 = Unbundle By Name(w866) -> ("Included?"=w868:bool)
          n471 = case shown="True" w868 {
            tunnel: w872 -> [w874 w899]
            tunnel: w871 -> [w873 w898]
            tunnel: [w874 w889] -> w870
            tunnel: [w873 w888] -> w869
            tunnel: w867 -> [_ w890]
            tunnel: w866 -> [_ w897]
            tunnel: w865 -> [_ w882]
            frame False {
              # "Saccade is not included. Do not export it."
            }
            frame True {
              # "Saccade is included. Export it."
              n472 = call <userlib>:"Write.vi"("error in (no error)"=w898, "Data"=w890, "Excel in"=w899) -> ("error out"=w887:errorcluster, "Last Cell"=w884:cluster{"Row":i32, "Col":i32}, "Excel out"=w886:refnum<class "Excel.lvclass">)  [unwired: 6 in]
              n473 = Unbundle By Name(w897) -> ("Impulse"=w891:i32, "Sequence #"=w879:dbl, "Onset (ms)"=w896:dbl, "Duration (ms)"=w895:dbl, "Vel (°/s)"=w894:dbl, "Amplitude (°)"=w893:dbl, "Gain"=w892:dbl)
              n474 = Add(x=w884, y=cluster{"Row":i32, "Col":i32} {"Row"=0, "Col"=1} ("Cell (Append to next row)")) -> (x+y=w883:cluster{"Row":i32, "Col":i32})
              n475 = To Double Precision Float(number=w891) -> (double precision float=w881:dbl)
              n476 = Build Array(w896, w895, w894, w893, w892) -> (w878:dbl[])
              n477 = Build Array (concatenate)(w882, w881, w879) -> (w880:dbl[])
              n478 = Number To Decimal String(number=w880) -> (decimal integer string=w877:string[])  [unwired: 1 in]
              n479 = Number To Fractional String(number=w878) -> (F-format string=w876:string[])  [unwired: 3 in]
              n480 = Build Array (concatenate)(w877, w876) -> (w875:string[])
              n481 = call <userlib>:"Write.vi"("error in (no error)"=w887, "Cell (Append to next row)"=w883, "Data"=w875, "Excel in"=w886) -> ("error out"=w888:errorcluster, "Excel out"=w889:refnum<class "Excel.lvclass">)  [unwired: 5 in, 1 out]
            }
          }
        }
        n482 = call <userlib>:"Save.vi"("error in (no error)"=w859, "Excel in"=w860) -> ("Excel out"=w858:refnum<class "Excel.lvclass">)  [unwired: 7 in, 2 out]
        n483 = Bundle By Name(cluster=w839, "Excel"=w858) -> (w841:T3)
      }
      frame "Do - Export All" {
        w901 = T10[] [enum."Export - Open Summary", enum."Export - Summary", enum."Export - Open Saccades", enum."Export - Saccades", enum."Export - Open Group", enum."Export - Group", enum."Give MCLB Focus"] items=["Initialise", "Quit", "DO - Analysis", "DO - Summary Analysis", "Load Channel Data", "Find Impulses", "Find Saccades", "Sequence Saccades", "Calc Saccade Summary Stats", "Calc Saccade Group Stats", "DO - Draw", "Clear Plot", "Plot Selected Saccade", "Plot Selected Saccade Siblings", "Plot Impulse Data", "Plot Saccade Data", "Fill Saccade MCLB", "Fill Summary Stats", "Give MCLB Focus", "Halt Panel Updates", "Resume Panel Updates", "Disable Controls", "Enable Controls", "Toggle Saccade", "DO - Export Summary", "Export - Open Summary", "Export - Summary", "DO - Export Saccades", "Export - Open Saccades", "Export - Saccades", "DO - Export Group", "Export - Open Group", "Export - Group", "Do - Export All"] ("element")
        # "Performs all Excel export options."
        n484 = for {
          tunnel: w900 -> [w906]
          tunnel: w901 -> [w905] mode=indexing
          n485 = Enqueue Element(queue=w906, element=w905) -> ()  [unwired: 2 in, 3 out]
        }
      }
    }
  }
  "Data OUT" <- w7
  "error out" <- w6
